vi "Martins HOT interface 120420.vi"() -> ()   [LabVIEW 2011]
uses:
  Sub VIs/Trap cluster.ctl
  <vilib>/Utility/inputDevices.llb/closeKeyboard.vi
  <vilib>/Utility/inputDevices.llb/keyboardAcquire.vi
  <vilib>/vision/driver/NI_Vision_Acquisition_Software.lvlib
  <vilib>/Utility/file.llb/Write To Spreadsheet File (DBL).vi
  <vilib>/vision/NI_Vision_Development_Module.lvlib
panel:
  in  "Apply Corrections":bool
  in  "View Licence":bool
  in  "ok":bool caption="Mark the center of \nthe spot using the \nzoom and the point\ntool, then click this \nbutton"
  in  "Stop program":bool
  in  "Updating trap cluster":bool=TRUE
  out "Camera enabled":bool=TRUE
  out "SLM enabled":bool=TRUE
  in  "Run calibration":bool
  in  "Hologram generation":cluster{"Method":i32, "Iterations":i32}={"Method"=1, "Iterations"=10} {"Method" items=["Lenses & Gratings (3D)", " Gerchberg-Saxton (3D)", "Gerchberg-Saxton FFT (2D)"]}
  in  "Display hologram\nand computed \nimage plane":bool
  in  "ROI":T1={"Global Rectangle"=[39, 191, 388, 192], "Contours"=[{"Contour Type"=0, "ROI Type"=1, "Points"=[387, 191]}, {"Contour Type"=0, "ROI Type"=1, "Points"=[300, 191]}, {"Contour Type"=0, "ROI Type"=1, "Points"=[213, 191]}, {"Contour Type"=0, "ROI Type"=1, "Points"=[126, 191]}, {"Contour Type"=0, "ROI Type"=1, "Points"=[39, 191]}]}
  out "Image":T2(plugin-control)
  out "Global Report":T3={"Mean Value"=79.60407, "Standard Variation"=8.375996, "Minimal Value"=27.0, "Maximal Value"=236.0, "Area (calibrated)"=180600.0, "Area (pixels)"=180600, "%"=100.0, "Calibration Valid"=TRUE} {"Mean Value" format="%.2f"; "%" format="%.2f"; "Area (calibrated)" format="%.2f"; "Maximal Value" format="%.2f"; "Minimal Value" format="%.2f"; "Standard Variation" format="%.2f"}
  in  "start path":path=path "E:/David/SLM characterization/Measured data/120420 - Trapping"
  in  "save image":bool
  in  "s":bool=TRUE
  in  "Edit trap cluster":bool
  out "Lost Frames":u32
  in  "threshold":bool=TRUE
  in  "Range":cluster{"Lower value":sgl, "Upper value":sgl}={"Lower value"=100.0, "Upper value"=255.0} {"Upper value" format="%.2f"; "Lower value" format="%.2f"}
  in  "Display data":bool
  in  "?":bool=TRUE
  in  "Follow traps":bool=TRUE
  in  "Purge data":bool
  in  "ROI size":dbl=54.0 min=2.0 step=2.0
  in  "Save data":bool
  in  "Video tracking":bool
  out "Calculated image plane":dbl[][](graph)
  in  "G":bool[](array[boolean])=[FALSE, FALSE, FALSE, FALSE, FALSE]
  out "Current trap pos":T4={"X (IMAQ)"=[387.0, 300.0, 213.0, 126.0, 39.0], "Y (IMAQ)"=[191.0, 191.0, 191.0, 191.0, 191.0], "Z"=[-28.0, -28.0, -28.0, -28.0, -28.0], "I"=[5.0, 5.0, 5.0, 5.0, 5.0], "Trap number"=[0, 1, 2, 3, 4], "ROI number"=[0, 1, 2, 3, 4], "Number of traps"=5, "Group"=[FALSE, FALSE, FALSE, FALSE, FALSE]}
  out "NI Vision error":errorcluster
  out "CUDA/SLM error":errorcluster
  in  "Cancel calibration":bool
  in  "Skip step if \ntimed out":bool
  in  "Display path":bool=TRUE
  out "Average step time (ms)":dbl=11.993055555555555
  in  "Step time \n(ms)":u32=10
  in  "Pause":bool
  in  "cancel path":bool
  out "Step skipped":bool
  in  "Path controls":T5={"follow path"=FALSE, "Step length"=1.0, "Arrive \nsimultaneously"=TRUE, "Synchronize traps"=FALSE, "Add current \npositions to path"=FALSE}
  in  "Create path":bool
  out "#":i32[](array[numeric])=[0, 1, 2, 3, 4]
  in  "Group \nTraps":bool
  in  "Move \nHandle":bool
  out "Displayed Hologram":u8[][](graph)
  in  "Coordinate mapping \n(IMAQ to SLM)":T6={"cZ"=1.0, "cY"=0.3667622, "cX"=-0.3678161, "sZ"=0.0, "sY"=-70.234955, "sX"=78.344826}
  in  "Switch X/Y":bool
  in  "I":dbl[](array[numeric])=[5.0, 5.0, 5.0, 5.0, 5.0]
  in  "Z":dbl[](array[numeric])=[-28.0, -28.0, -28.0, -28.0, -28.0]
  in  "Max num of \nmeasurements":i32=-1
  # "Martin\nPersson 2011"
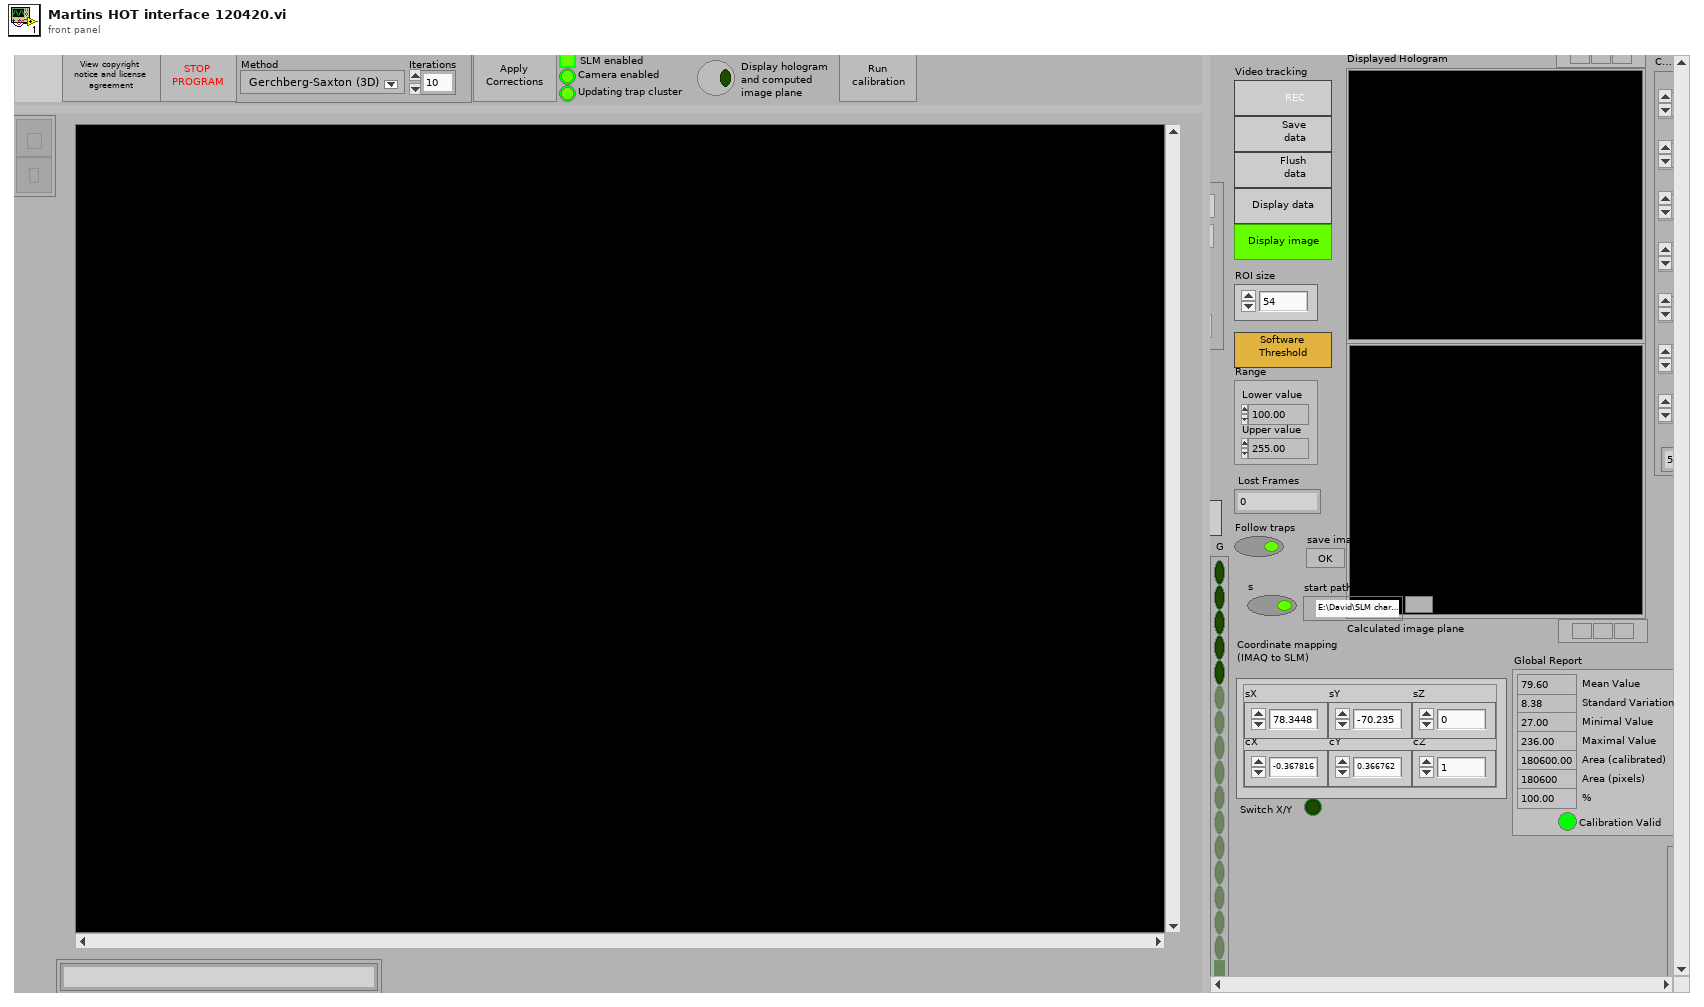
[diagram p1: front panel]
types:
  T1 = cluster{"Global Rectangle":i32[], "Contours":cluster{"Contour Type":u32, "ROI Type":u32, "Points":i32[]}[]}
  T2 = typedef "IMAQ Image.ctl" = refnum<image>
  T3 = cluster{"Mean Value":sgl, "Standard Variation":sgl, "Minimal Value":sgl, "Maximal Value":sgl, "Area (calibrated)":sgl, "Area (pixels)":u32, "%":sgl, "Calibration Valid":bool}
  T4 = typedef "Trap cluster.ctl" = cluster{"X (IMAQ)":sgl[], "Y (IMAQ)":sgl[], "Z":sgl[], "I":sgl[], "Trap number":i32[], "ROI number":i32[], "Number of traps":i32, "Group":bool[]}
  T5 = cluster{"follow path":bool, "Step length":dbl, "Arrive \nsimultaneously":bool, "Synchronize traps":bool, "Add current \npositions to path":bool}
  T6 = cluster{"cZ":sgl, "cY":sgl, "cX":sgl, "sZ":sgl, "sY":sgl, "sX":sgl}
  T7 = cluster{"Centroid X":dbl[], "Centroid Y":dbl[], "Acquired Buffer Number":u32}
  T8 = typedef "IMAQdx.ctl" = refnum<k21>
  T9 = typedef "Image Type" = u32
  T10 = enum16{"0", "1", "2", "3", "4", "5", "6", "7", "8", "9", "A", "B", "C", "D", "E", "F", "G", "H", "I", "J", "K", "L", "M", "N", "O", "P", "Q", "R", "S", "T", "U", "V", "W", "X", "Y", "Z", "F1", "F2", "F3", "F4", "F5", "F6", "F7", "F8", "F9", "F10", "F11", "F12", "F13", "F14", "F15", "ADD", "BACK", "BACKSLASH", "CAPITAL", "COMMA", "DECIMAL", "DELETE", "DIVIDE", "DOWN", "END", "EQUALS", "ESCAPE", "GRAVE (`)", "HOME", "INSERT", "LBRACKET", "LCONTROL", "LEFT", "L ALT", "LSHIFT", "LWIN", "MINUS", "MULTIPLY", "NEXT", "NUMLOCK", "NUMPAD_0", "NUMPAD_1", "NUMPAD_2", "NUMPAD_3", "NUMPAD_4", "NUMPAD_5", "NUMPAD_6", "NUMPAD_7", "NUMPAD_8", "NUMPAD_9", "PAUSE", "PERIOD", "PRIOR (PG UP)", "RBRACKET", "RCONTROL", "RETURN", "RIGHT", "R ALT", "RSHIFT", "RWIN", "SCROLL", "SEMICOLON", "SLASH", "SPACE", "SUBTRACT", "TAB", "UP", "ENTER (num pad)", "' (quote)"}[]
  T11 = typedef "LVRectTypeDef.ctl" = cluster{"left":i16, "top":i16, "right":i16, "bottom":i16}
  T12 = cluster{"CentroidX":dbl[], "CentroidY":dbl[], "Acquired Buffer Number":u32}
  T13 = cluster{"Centroid X":dbl[], "Centroid Y":dbl[], "Acquired Buffer Number":u32}[]
  T14 = cluster{"Contour Type":u32, "ROI Type":u32, "Points":i32[]}[]
  T15 = cluster{"Contour Type":u32, "ROI Type":u32, "Points":i32[]}
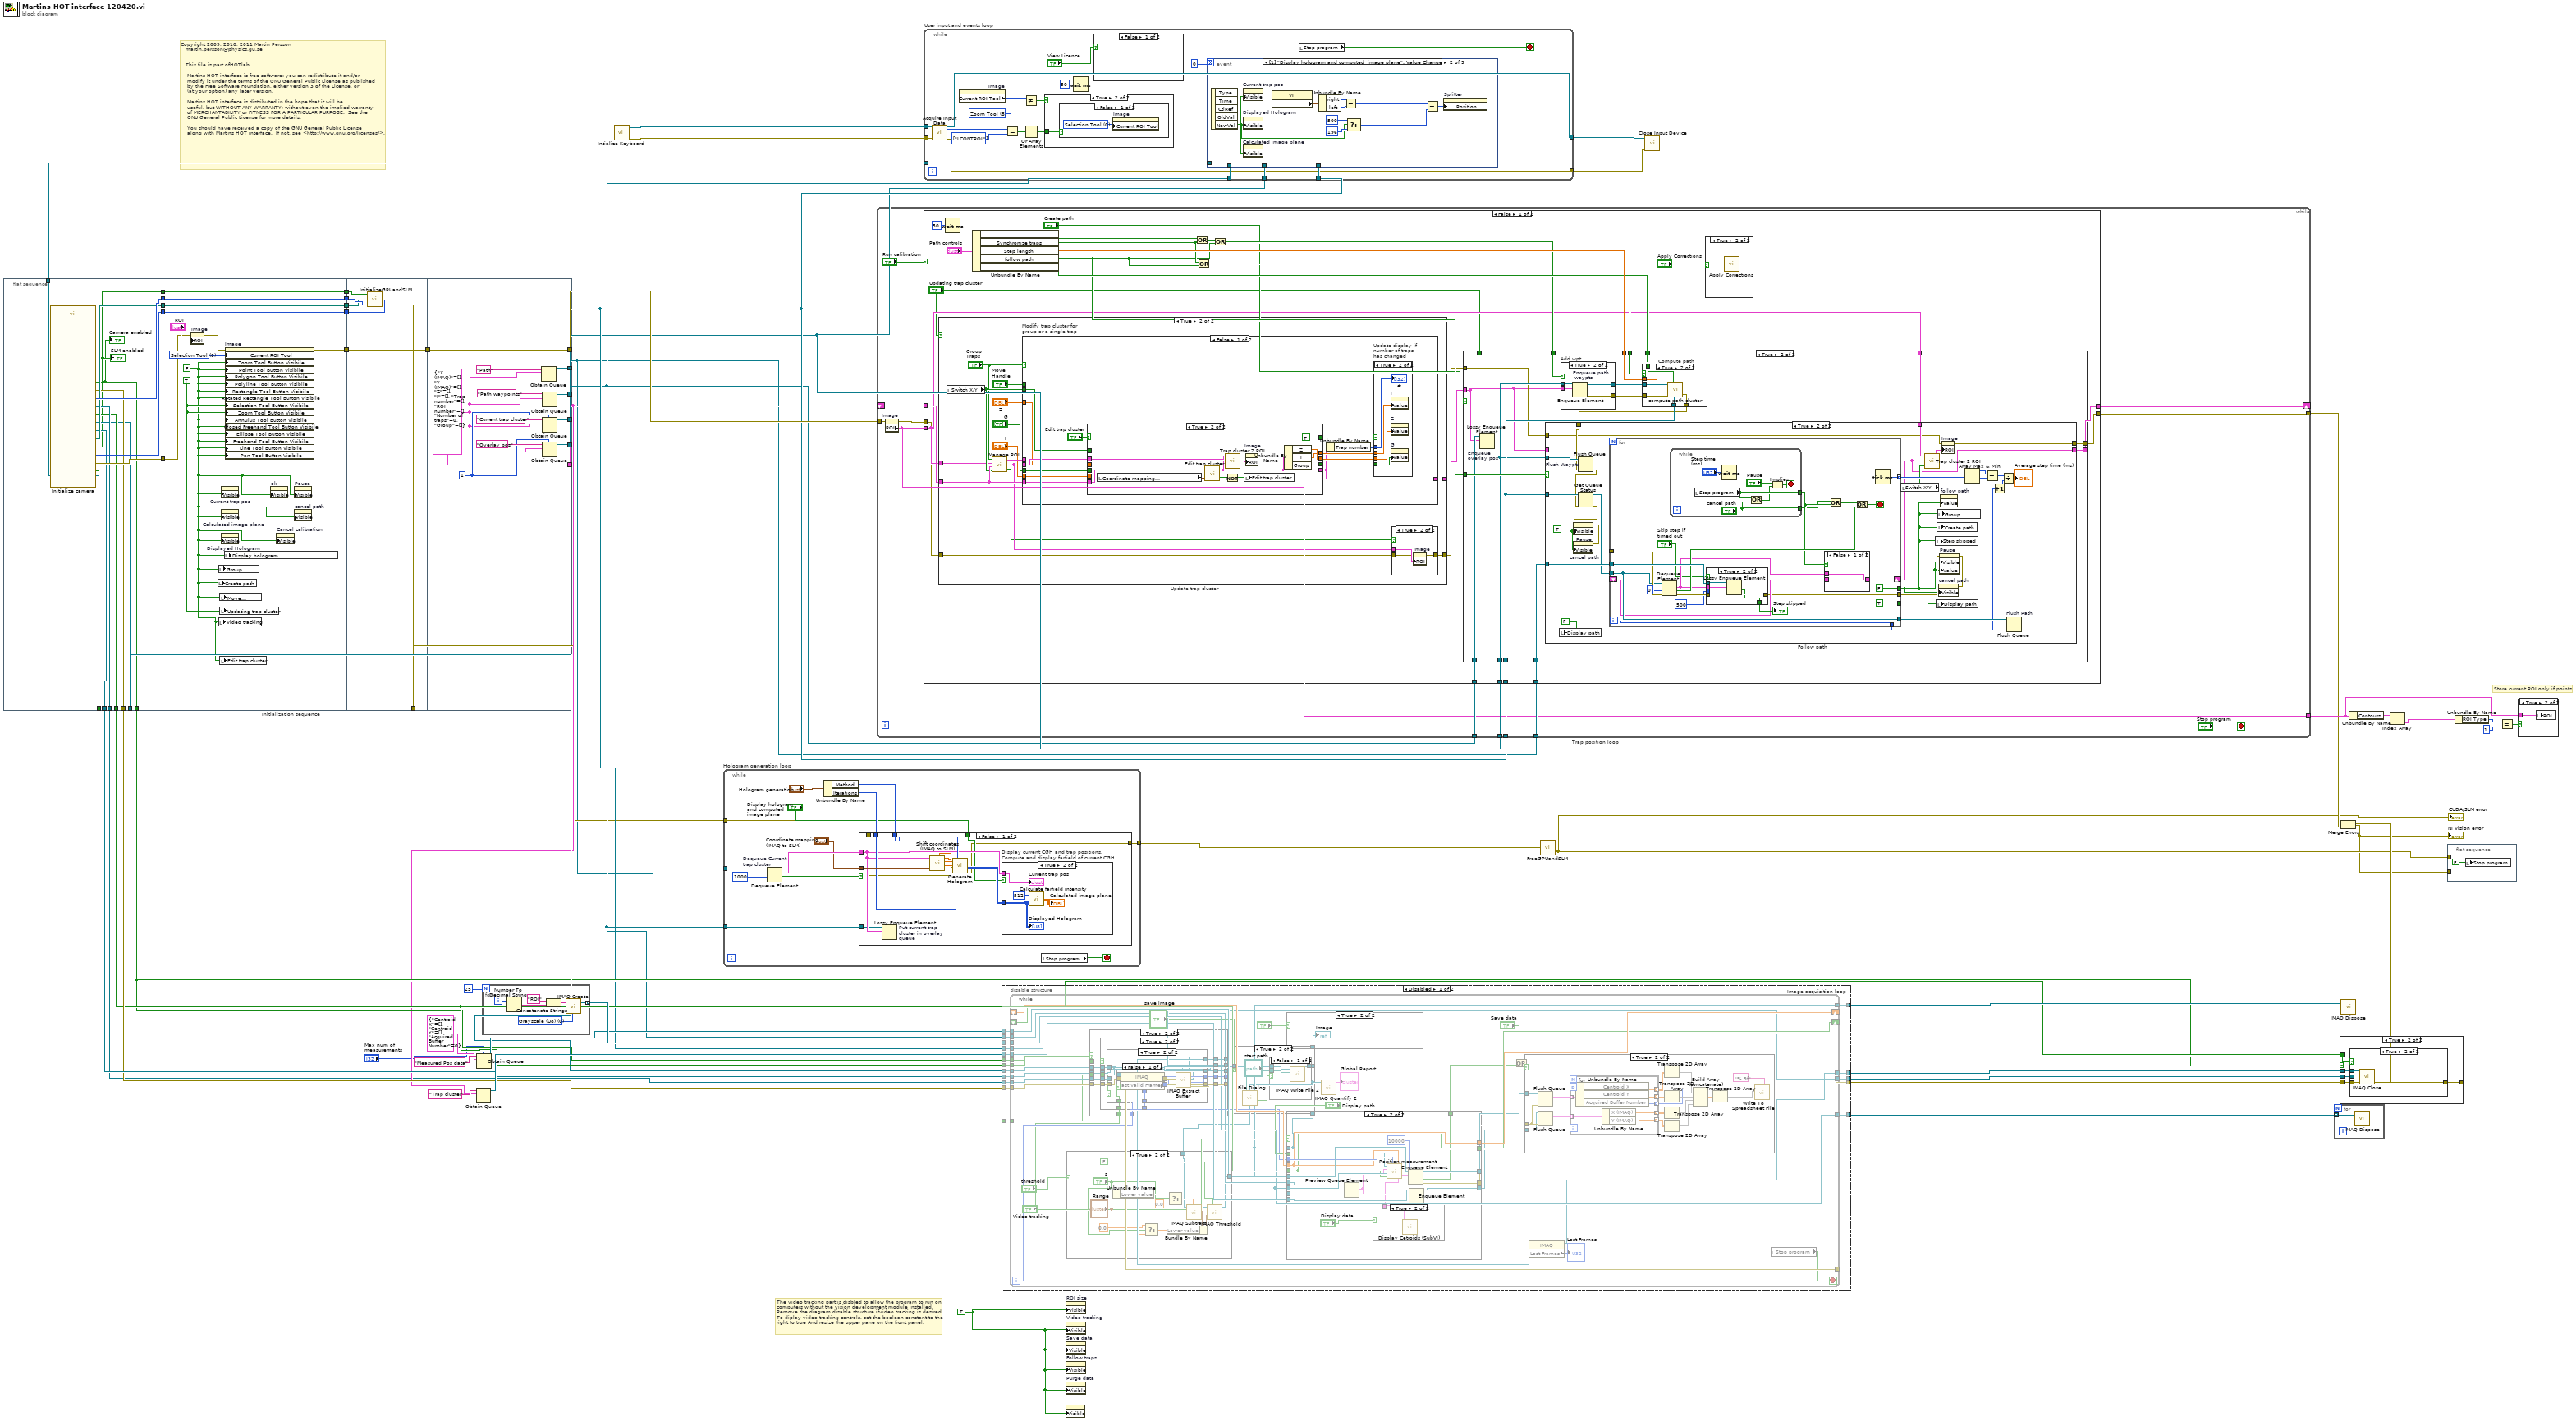
[diagram p0: block diagram]
diagram:
  w42 = TRUE ("Visible")
  # "Copyright 2009, 2010, 2011 Martin Persson \n   martin.persson@physics.gu.se\n\n\n   This file is part ofHOTlab.\n\n    Martins HOT interface is free software: you can redistribute it and/or \n    modify it under the terms of the GNU General Public License as published \n    by the Free Software Foundation, either version 3 of the License, or\n    (at your option) any later version.\n\n    Martins HOT interface is distributed in the hope that it will be \n    useful, but WITHOUT ANY WARRANTY; without even the implied warranty\n    of MERCHANTABILITY or FITNESS FOR A PARTICULAR PURPOSE.  See the\n    GNU General Public License for more details.\n\n    You should have received a copy of the GNU General Public License\n    along with Martins HOT interface.  If not, see <http://www.gnu.org/licenses/>."
  # "Store current ROI only if points"
  # "The video tracking part is disbled to allow the program to run on\ncomputers without the vision development module installed. \nRemove the diagram disable structure ifvideo tracking is desired. \nTo diplay video tracking controls, set the boolean constant to the \nright to true And resize the upper pane on the front panel."
  n1 = flat-sequence "Initialization sequence" {
    tunnel: [w59] -> w28
    tunnel: [w68] -> w27
    tunnel: [w67] -> w26
    tunnel: [w66] -> w25
    tunnel: [w65] -> w24
    tunnel: [w64] -> w4
    tunnel: [w63] -> w22
    tunnel: [w62] -> w21
    tunnel: [w61] -> w20
    tunnel: [w60] -> w19
    tunnel: [w58] -> w18
    tunnel: [w57] -> w5
    tunnel: [w56] -> w3
    tunnel: w28 -> [w76]
    tunnel: w27 -> [w74]
    tunnel: w26 -> [w79]
    tunnel: w25 -> [w78]
    tunnel: w24 -> [w77]
    tunnel: [w76] -> w13
    tunnel: [w71] -> w12
    tunnel: [w79] -> w10
    tunnel: [w78] -> w9
    tunnel: [w77] -> w8
    tunnel: w13 -> [w82]
    tunnel: w12 -> [w85]
    tunnel: [w85] -> w11
    tunnel: w10 -> [w83]
    tunnel: w9 -> [w84]
    tunnel: w8 -> [w81]
    tunnel: [w80] -> w7
    tunnel: [w96] -> w23
    tunnel: w11 -> [w96]
    tunnel: [w94] -> w17
    tunnel: [w92] -> w16
    tunnel: [w90] -> w6
    tunnel: [w89] -> w15
    tunnel: [w86] -> w14
    frame #0 {
      n2 = call "Initialize camera.vi"() -> ("CUDA device ID"=w66:i32, "IMAQdx Session Out"=w63:T8, "TrueFrame out"=w67:i32, "IMAQ camera"=w61:bool, "Image buffers"=w56:T2[], "Image reference out"=w64:T2, "Ring?"=w57:bool, "SLM enabled"=w59:bool, "Camera enabled"=w58:bool, "Vision error out"=w68:errorcluster, "LUT path out"=w65:path, "IMAQ Session Out"=w60:refnum<k11>, "Camera error"=w62:errorcluster)  [unwired: 3 in]
      "Camera enabled" <- w58
      "SLM enabled" <- w59
    }
    frame #1 {
      w70 = TRUE ("ROI Tool Buttons Visibile:Zoom Tool Button Visible")
      w69 = FALSE ("ROI Tool Buttons Visibile:Zoom Tool Button Visible")
      w73 = u32 0 items=["Zoom Tool"=8, "Selection Tool"=0, "Pan Tool"=9, "Point Tool"=1, "Line Tool"=2, "Rectangle Tool"=3, "Rotated Rectangle Tool"=12, "Polyline Tool"=10, "Polygon Tool"=5, "Freehand Tool"=11, "Closed Freehand Tool"=6, "Ellipse Tool"=4, "Annulus Tool"=7] ("Current ROI Tool")
      n3 = property on="Image" class="ImageControl"(error in=w74, "ROI"="ROI") -> (error out=w72:errorcluster)  [unwired: 1 in, 1 out]
      n4 = local write "Create path"(w69) -> ()
      n5 = local write "Group \nTraps"(w69) -> ()
      n6 = local write "Video tracking"(w69) -> ()
      n7 = local write "Move \nHandle"(w69) -> ()
      n8 = local write "Updating trap cluster"(w70) -> ()
      n9 = local write "Edit trap cluster"(w69) -> ()
      n10 = property on="Current trap pos" class="Clust (strict)"("Visible"=w69) -> ()  [unwired: 2 in, 2 out]
      n11 = property on="Calculated image plane" class="IntGraph (strict)"("Visible"=w69) -> ()  [unwired: 2 in, 2 out]
      n12 = property on="Displayed Hologram" class="IntGraph (strict)"("Visible"=w69) -> ()  [unwired: 2 in, 2 out]
      n13 = local write "Display hologram\nand computed \nimage plane"(w69) -> ()
      n14 = property on="Image" class="ImageControl"(error in=w72, "Current ROI Tool"=w73, "Zoom Tool Button Visibile"=w69, "Point Tool Button Visibile"=w69, "Polygon Tool Button Visibile"=w69, "Polyline Tool Button Visibile"=w69, "Rectangle Tool Button Visibile"=w69, "Rotated Rectangle Tool Button Visibile"=w69, "Selection Tool Button Visibile"=w70, "Zoom Tool Button Visibile"=w70, "Annulus Tool Button Visibile"=w69, "Closed Freehand Tool Button Visibile"=w69, "Ellipse Tool Button Visibile"=w69, "Freehand Tool Button Visibile"=w69, "Line Tool Button Visibile"=w69, "Pan Tool Button Visibile"=w69) -> (error out=w71:errorcluster)  [unwired: 1 in, 1 out]
      n15 = property on="ok" class="Bool"("Visible"=w69) -> ()  [unwired: 2 in, 2 out]
      n16 = property on="Cancel calibration" class="Bool"("Visible"=w69) -> ()  [unwired: 2 in, 2 out]
      n17 = property on="Pause" class="Bool (strict)"("Visible"=w69) -> ()  [unwired: 2 in, 2 out]
      n18 = property on="cancel path" class="Bool"("Visible"=w69) -> ()  [unwired: 2 in, 2 out]
    }
    frame #2 {
      n19 = call "InitializeGPUandSLM.vi"("TrueFrame"=w83, "deviceId"=w84, "Path to LUT file"=w81, "SLM enabled"=w82) -> ("CUDA/SLM error"=w80:errorcluster)  [unwired: 1 out]
    }
    frame #3 {
      w87 = 1 ("max queue size (-1, unlimited)")
      w86 = T4 {"X (IMAQ)"=[], "Y (IMAQ)"=[], "Z"=[], "I"=[], "Trap number"=[], "ROI number"=[], "Number of traps"=0, "Group"=[]} ("output cluster 2")
      n20 = Obtain Queue(name (unnamed)="Path", element data type=w86) -> (queue out=w94:refnum<queue>)  [unwired: 3 in, 2 out]
      n21 = Obtain Queue(name (unnamed)="Path waypoints", element data type=w86) -> (queue out=w92:refnum<queue>)  [unwired: 3 in, 2 out]
      n22 = Obtain Queue(max queue size (-1, unlimited)=w87, name (unnamed)="Current trap cluster", element data type=w86) -> (queue out=w90:refnum<queue>)  [unwired: 2 in, 2 out]
      n23 = Obtain Queue(max queue size (-1, unlimited)=w87, name (unnamed)="Overlay pos", element data type=w86) -> (queue out=w89:refnum<queue>)  [unwired: 2 in, 2 out]
    }
  }
  n24 = Obtain Queue(name (unnamed)="Trap cluster", element data type=w14) -> (queue out=w47:refnum<queue>)  [unwired: 3 in, 2 out]
  n25 = Obtain Queue(max queue size (-1, unlimited)="Max num of \nmeasurements", name (unnamed)="Measured Pos data", element data type=T7 {"Centroid X"=[], "Centroid Y"=[], "Acquired Buffer Number"=0} ("output cluster 2")) -> (queue out=w50:refnum<queue>)  [unwired: 2 in, 2 out]
  n26 = for {
    N: 25 -> [_]
    tunnel: [w102] -> w52 mode=indexing
    i -> [w98]
    w100 = T9 0 items=["Grayscale (U8)", "Grayscale (I16)", "Grayscale (SGL)", "Complex (CSG)", "RGB (U32)", "HSL (U32)", "RGB (U64)", "Grayscale (U16)"] ("Image Type")
    n27 = Number To Decimal String(number=w98) -> (decimal integer string=w97:string)  [unwired: 1 in]
    n28 = Concatenate Strings("ROI" ("Image Name"), w97) -> (w99:string)
    n29 = call "IMAQ Create"("Image Name"=w99, "Image Type"=w100) -> ("New Image"=w102:T2)  [unwired: 3 in, 1 out]
  }
  n30 = call <vilib>:"Intialize Keyboard.vi"() -> ("error out"=w30:errorcluster, "device ID"=w55:refnum<k1>)  [unwired: 1 in, 9 out]
  n31 = while "Hologram generation loop" {
    tunnel: w6 -> [w111]
    tunnel: w15 -> [w109]
    tunnel: w7 -> [w104]
    tunnel: [w103] -> w1
    stop <- w112 stop-if-true
    n32 = Dequeue Element "Dequeue Current \ntrap cluster"(queue=w111, timeout in ms (-1)=1000) -> (element=w110:T4, timed out?=w108:bool)  [unwired: 1 in, 2 out]
    n33 = Unbundle By Name("Hologram generation") -> ("Method"=w115:i32, "Iterations"=w114:i32)
    n34 = case shown="False" w108 {
      tunnel: "Coordinate mapping \n(IMAQ to SLM)" -> [w128 _]
      tunnel: "Display hologram\nand computed \nimage plane" -> [w118 _]
      tunnel: w115 -> [w122 _]
      tunnel: w114 -> [w121 _]
      tunnel: w110 -> [w120 _]
      tunnel: w109 -> [w119 _]
      tunnel: w104 -> [w117 w133]
      tunnel: [w116 w133] -> w103
      frame False {
        n35 = Lossy Enqueue Element "Put current trap \ncluster in overlay \nqueue"(queue=w119, element=w120) -> ()  [unwired: 1 in, 4 out]
        n36 = call "Shift coordinates (IMAQ to SLM).vi"("Trap cluster"=w120, "Coordinate mapping \n(IMAQ to SLM)"=w128) -> ("X (SLM)"=w123:sgl[], "Y (SLM)"=w126:sgl[], "Intensities"=w124:sgl[], "Z (SLM)"=w125:sgl[])  [unwired: 1 in, 1 out]
        n37 = call "Generate Hologram.vi"("x"=w123, "y"=w126, "z"=w125, "spot_intensities"=w124, "CUDA/SLM error in"=w117, "N_iterations"=w121, "method"=w122) -> ("CGH out"=w127:u8[][], "CUDA/SLM error out"=w116:errorcluster)  [unwired: 17 in, 2 out]
        n38 = case "Display current CGH and trap positions.\nCompute and display farfield of current CGH" shown="True" w118 {
          tunnel: w127 -> [_ w131]
          tunnel: w120 -> [_ w130]
          frame False {
          }
          frame True {
            n39 = call "Calculate farfield intensity.vi"("h_pSLM"=w131, "SLMsize"=512 ("Numeric")) -> ("Calculated image plane"=→"Calculated image plane":dbl[][])
            "Displayed Hologram" <- w131
            "Current trap pos" <- w130
          }
        }
      }
      frame True {
      }
    }
    n40 = local read "Stop program"() -> (w112:bool)
  }
  n41 = while "Trap position loop" {
    tunnel: w16 -> [w145]
    tunnel: w17 -> [w142]
    shift-right: [w144] -> _
    shift-left: w14 -> [w137]
    tunnel: w6 -> [w143]
    tunnel: w15 -> [w140]
    tunnel: [w139] -> w36
    tunnel: w23 -> [w136]
    tunnel: [w134] -> w34
    stop <- "Stop program" stop-if-true
    n42 = property on="Image" class="ImageControl"(error in=w136) -> (error out=w135:errorcluster, "ROI"=w139:T1)  [unwired: 1 in, 1 out]
    n43 = case shown="False" "Run calibration" {
      selector: "Run calibration" -> [_ w346]
      tunnel: w145 -> [w169 _]
      tunnel: w137 -> [w168 w345]
      tunnel: [w147 w345] -> w144
      tunnel: w143 -> [w158 w355]
      tunnel: w142 -> [w156 _]
      tunnel: w140 -> [w153 _]
      tunnel: w139 -> [w152 w354]
      tunnel: w135 -> [w151 w350]
      tunnel: [w149 w347] -> w134
      frame False {
        n44 = case "Update trap cluster" shown="True" "Updating trap cluster" {
          tunnel: w168 -> [w171 w185]
          tunnel: [w171 w178] -> w159
          tunnel: w152 -> [_ w176]
          tunnel: w151 -> [w170 w175]
          tunnel: [w170 w174] -> w150
          frame False {
          }
          frame True {
            n45 = local read "Switch X/Y"() -> (w184:bool)
            n46 = call "Manage ROI.vi"("Switch X/Y"=w184, "Trap cluster in"=w185, "ROI in"=w176, "Group traps"="Group \nTraps") -> ("Replace ROI"=w172:bool, "ROI out"=w177:T1, "Previous ROI out"=w183:T1)
            n47 = case "Modify trap cluster for \ngroup or a single trap" shown="False" "Group \nTraps" {
              tunnel: [w195 w234] -> w178
              tunnel: w177 -> [w202 w235]
              tunnel: w185 -> [w201 w237]
              tunnel: w183 -> [_ w236]
              tunnel: "Z" -> [w200 w233]
              tunnel: "Move \nHandle" -> [_ w232]
              tunnel: w184 -> [w199 w231]
              tunnel: "I" -> [w197 w230]
              tunnel: "G" -> [w192 w229]
              frame False {
                n48 = case shown="True" "Edit trap cluster" {
                  tunnel: w202 -> [w213 w216]
                  tunnel: w201 -> [w212 w224]
                  tunnel: w200 -> [w211 _]
                  tunnel: w199 -> [w210 _]
                  tunnel: [w209 w223] -> w198
                  tunnel: w197 -> [w208 _]
                  tunnel: [w207 w222] -> w196
                  tunnel: [w206 w218] -> w195
                  tunnel: [w205 TRUE ("Update display")] -> w193
                  tunnel: w192 -> [w204 _]
                  tunnel: [w203 w220] -> w191
                  frame False {
                    n49 = call "ROI 2 Trap Cluster.vi"("Amplitudes"=w208, "Switch X/Y"=w210, "Group"=w204, "Trap Cluster in"=w212, "Z"=w211, "ROI"=w213) -> ("Group out"=w203:bool[], "Z out"=w209:dbl[], "Amplitudes out"=w207:dbl[], "Trap Cluster Out"=w206:T4, "Update display"=w205:bool)
                  }
                  frame True {
                    n50 = local read "Coordinate mapping \n(IMAQ to SLM)"() -> (w215:T6)
                    n51 = call "Edit trap cluster.vi"("Coordinate mapping \n(IMAQ to SLM)"=w215, "trap cluster in"=w224) -> ("SubVI closed"=w219:bool, "Trap cluster out"=w218:T4)
                    n52 = Not(x=w219) -> (.not. x?=w214:bool)
                    n53 = call "Trap cluster 2 ROI.vi"("Trap cluster"=w218, "ROI in"=w216) -> ("ROI out"=w217:T1)  [unwired: 1 in]
                    n54 = local write "Edit trap cluster"(w214) -> ()
                    n55 = property on="Image" class="ImageControl"("ROI"=w217) -> ()  [unwired: 2 in, 2 out]
                    n56 = Unbundle By Name(w218) -> ("Z"=w223:sgl[], "I"=w222:sgl[], "Group"=w220:bool[])
                  }
                }
                n57 = Unbundle By Name(w195) -> ("Trap number"=w194:i32[])
                n58 = case "Update display if\nnumber of traps \nhas changed" shown="True" w193 {
                  tunnel: w198 -> [_ w228]
                  tunnel: w196 -> [_ w227]
                  tunnel: w194 -> [_ w226]
                  tunnel: w191 -> [_ w225]
                  frame False {
                  }
                  frame True {
                    n59 = property on="I" class="Arr (strict)"("Value"=w227) -> ()  [unwired: 2 in, 2 out]
                    n60 = property on="Z" class="Arr (strict)"("Value"=w228) -> ()  [unwired: 2 in, 2 out]
                    n61 = property on="G" class="Arr (strict)"("Value"=w225) -> ()  [unwired: 2 in, 2 out]
                    "#" <- w226
                  }
                }
              }
              frame True {
                n62 = call "Move group.vi"("New handle position in"=w235, "Trap cluster in"=w237, "Previous handle position in"=w236, "Amplitudes"=w230, "Group"=w229, "Switch X/Y"=w231, "Move handle"=w232, "Z"=w233) -> ("Trap cluster out"=w234:T4)
              }
            }
            n63 = case shown="True" w172 {
              tunnel: w177 -> [_ w189]
              tunnel: w175 -> [w186 w188]
              tunnel: [w186 w187] -> w174
              frame False {
              }
              frame True {
                n64 = property on="Image" class="ImageControl"(error in=w188, "ROI"=w189) -> (error out=w187:errorcluster)  [unwired: 1 in, 1 out]
              }
            }
          }
        }
        n65 = Wait (ms)(milliseconds to wait=u32 50) -> ()  [unwired: 1 out]
        n66 = Unbundle By Name("Path controls") -> ("Add current \npositions to path"=w154:bool, "Synchronize traps"=w163:bool, "Step length"=w166:dbl, "follow path"=w157:bool, "Arrive \nsimultaneously"=w165:bool)
        n67 = Or(x=w154, y=w163) -> (x .or. y?=w164:bool)
        n68 = Or(x=w163, y=w157) -> (x .or. y?=w161:bool)
        n69 = Or(x=w164, y=w157) -> (x .or. y?=w162:bool)
        n70 = case shown="True" "Create path" {
          tunnel: w169 -> [_ w250]
          tunnel: w159 -> [w238 w244]
          tunnel: w166 -> [_ w259]
          tunnel: w156 -> [_ w254]
          tunnel: w165 -> [_ w258]
          tunnel: w162 -> [_ w257]
          tunnel: w161 -> [_ w256]
          tunnel: w157 -> [_ w255]
          tunnel: w158 -> [w241 w251]
          tunnel: w153 -> [_ w249]
          tunnel: w152 -> [_ w248]
          tunnel: w150 -> [w240 w247]
          tunnel: [w240 w246] -> w149
          tunnel: "Updating trap cluster" -> [w239 _]
          tunnel: [w238 w245] -> w147
          frame False {
            n71 = case shown="True" w239 {
              tunnel: w238 -> [_ w243]
              tunnel: w241 -> [_ w242]
              frame False {
              }
              frame True {
                n72 = Lossy Enqueue Element(queue=w242, element=w243) -> ()  [unwired: 1 in, 4 out]
              }
            }
          }
          frame True {
            n73 = Lossy Enqueue Element "Enqueue\noverlay pos"(queue=w249, element=w244) -> ()  [unwired: 1 in, 4 out]
            n74 = case "Add wpt" shown="True" w257 {
              tunnel: w244 -> [_ w336]
              tunnel: w250 -> [w333 w337]
              tunnel: [w333 w334] -> w260
              tunnel: [_ w335] -> w252
              frame False {
              }
              frame True {
                n75 = Enqueue Element "Enqueue path\n waypts"(queue=w337, element=w336) -> (queue out=w334:refnum<queue>, error out=w335:errorcluster)  [unwired: 2 in, 1 out]
              }
            }
            n76 = case "Compute path" shown="True" w256 {